vi "SNR_output.vi"() -> ()   [LabVIEW 2019]
uses:
  MeasSNRResults.ctl
  <vilib>/imath/engines/lvmath2/RunTimeEngine/Managers/WorkSpace/UID Generator.vi
  <vilib>/imath/engines/lvmath2/RunTimeEngine/RunTimeType/NIMS_RunTimeType_From StrictType (excl LVString).vi
  <instcachedir>/0/NIMS_RunTimeType_From StrictType (excl LVString)_D8AFBA86A94845AAA577C895450664BD.lvgen/NIMS_RunTimeType_From StrictType (excl LVString)_D8AFBA86A94845AAA577C895450664BD_000.vi
  <vilib>/imath/engines/lvmath2/RunTimeEngine/LocalVariableDefStatement/MC_LocalVariableDefStatement_Display.vi
  <vilib>/imath/engines/lvmath2/RunTimeEngine/Managers/SymbolTable/Clear UID.vi
  <vilib>/imath/engines/lvmath2/RunTimeEngine/NodeEndStatement/NIMS_NodeEndStatement_Output.vi
  <instcachedir>/0/NIMS_NodeEndStatement_Output_53EC0D466D134D7ABD903AC30B43404B.lvgen/NIMS_NodeEndStatement_Output_53EC0D466D134D7ABD903AC30B43404B_009.vi
  <instcachedir>/0/NIMS_NodeEndStatement_Output_53EC0D466D134D7ABD903AC30B43404B.lvgen/NIMS_NodeEndStatement_Output_53EC0D466D134D7ABD903AC30B43404B_001.vi
  <vilib>/imath/engines/lvmath2/RunTimeEngine/ErrorHandling/NIMS_Finalize Error.vi
  <vilib>/measure/NI_MABase.lvlib
  <vilib>/imath/engines/lvmath2/RunTimeEngine/Managers/SymbolTable/NIMS_WorkSpace.lvlib
panel:
  in  "Tab Control":enum32{"Part 1", "Part 2", "Part 3", "Part 4"}(tab)=enum."Part 4"
  in  "standard deviation":dbl=0.1 format="%.2p"
  in  "amplitude":dbl=1.0 format="%0.2p"
  in  "frequency":dbl=1001.0 format="%0.2p"
  in  "VRef":dbl=1.0
  in  "LowerNoiseBW":dbl
  in  "IgnoreDC":bool
  in  "sampling info":cluster{"Fs":dbl, "#s":dbl}={"Fs"=100000.0, "#s"=20000.0} {"Fs" format="%.2p"}
  out "MeasSNRResults":T1={"VSignalRMS"=0.7053309596420384, "VNoiseRMS"=0.09844196981459605, "SNR(dB)"=17.10425303559703, "NumBits"=2.548879241793527, "SNRFS(dB)"=17.12609413716782, "NumBitsFS"=2.552507331755452} {"SNRFS(dB)" format="%_3p"; "NumBitsFS" format="%.1f"; "NumBits" format="%.1f"; "SNR(dB)" format="%_3p"; "VNoiseRMS" format="%#_3p"; "VSignalRMS" format="%#_3p"}
  out "Input":waveform(dbl)(graph)={"t0"=timestamp(0 s since 1904-01-01), "dt"=1e-05, "Y"=array[20000 elements]} caption="Histogram"
  out "MeasSNR Expected":T1={"VSignalRMS"=0.7071067811865475, "VNoiseRMS"=0.1, "SNR(dB)"=16.989700043360187, "NumBits"=2.5298505055415594, "SNRFS(dB)"=16.989700043360187, "NumBitsFS"=2.8200236127281304} {"SNRFS(dB)" format="%_3p"; "NumBitsFS" format="%.1f"; "NumBits" format="%.1f"; "SNR(dB)" format="%_3p"; "VNoiseRMS" format="%#_3p"; "VSignalRMS" format="%#_3p"}
  out "UpperNoiseBW":dbl=50000.0
  out "Mag Spectrum 1":cluster{"f0":dbl, "df":dbl, "magnitude":dbl[]}(graph)={"f0"=0.0, "df"=5.0, "magnitude"=array[10000 elements]} caption="Histogram"
  in  "IgnoreDC 2":bool=TRUE
  in  "LowerNoiseBW 2":dbl
  in  "VRef 2":dbl=1.0
  in  "sampling info 2":cluster{"Fs":dbl, "#s":dbl}={"Fs"=100000.0, "#s"=20000.0} {"Fs" format="%.2p"}
  out "Input 2":waveform(dbl)(graph)={"t0"=timestamp(2.8000000000000003 s since 1904-01-01), "dt"=1e-05, "Y"=array[20000 elements]} caption="Histogram"
  in  "amplitude 2":dbl=1.0 format="%0.2p"
  in  "frequency 2":dbl=1001.0 format="%0.2p"
  out "delta":dbl=7.62939453125e-06
  out "sigma":dbl=2.2024164931855234e-06
  out "MeasSNRResults 2":T1={"VSignalRMS"=0.7071067986176297, "VNoiseRMS"=2.453932856011485e-06, "SNR(dB)"=109.19244674787093, "NumBits"=17.845921386689525, "SNRFS(dB)"=109.1924465337527, "NumBitsFS"=17.84592135112171} {"SNRFS(dB)" format="%_3p"; "NumBitsFS" format="%.1f"; "NumBits" format="%.1f"; "SNR(dB)" format="%_3p"; "VNoiseRMS" format="%#_3p"; "VSignalRMS" format="%#_3p"}
  out "2^(N-1)/Vref":dbl=131072.0
  out "Results: Bits 4-18":T1[](array[typedef])=[{"VSignalRMS"=0.7101470628693265, "VNoiseRMS"=0.038700707438026845, "SNR(dB)"=25.272587825922308, "NumBits"=3.905745486033606, "SNRFS(dB)"=25.235321965915688, "NumBitsFS"=3.899555143839815}, {"VSignalRMS"=0.7082317616189774, "VNoiseRMS"=0.019483292047133716, "SNR(dB)"=31.210261178048867, "NumBits"=4.892069963131041, "SNRFS(dB)"=31.196453233668976, "NumBitsFS"=4.889776284662621}, {"VSignalRMS"=0.7074174458063527, "VNoiseRMS"=0.009851316989764243, "SNR(dB)"=37.12362944196923, "NumBits"=5.874357050161002, "SNRFS(dB)"=37.119814168121, "NumBitsFS"=5.873723283741032}, {"VSignalRMS"=0.707070558192555, "VNoiseRMS"=0.0049426927430694465, "SNR(dB)"=43.109982802020106, "NumBits"=6.868767907312311, "SNRFS(dB)"=43.11042776591464, "NumBitsFS"=6.8688418215805065}, {"VSignalRMS"=0.7071264669443802, "VNoiseRMS"=0.0024726949970293767, "SNR(dB)"=49.12653085128376, "NumBits"=7.868194493568732, "SNRFS(dB)"=49.126289040648615, "NumBitsFS"=7.868154325689139}, {"VSignalRMS"=0.707117724944963, "VNoiseRMS"=0.0012448255565093345, "SNR(dB)"=55.08766455446092, "NumBits"=8.858416038946999, "SNRFS(dB)"=55.087530125623886, "NumBitsFS"=8.858393708575397}, {"VSignalRMS"=0.7071124254509354, "VNoiseRMS"=0.0006223588128025631, "SNR(dB)"=61.108952501973235, "NumBits"=9.858629983716485, "SNRFS(dB)"=61.10888316978296, "NumBitsFS"=9.858618466741357}, {"VSignalRMS"=0.7071037089140556, "VNoiseRMS"=0.00031251710643333074, "SNR(dB)"=67.09218641311259, "NumBits"=10.85252265998548, "SNRFS(dB)"=67.09222415207716, "NumBitsFS"=10.852528928916472}, {"VSignalRMS"=0.7071095465375292, "VNoiseRMS"=0.00015693733289259758, "SNR(dB)"=73.07520865966347, "NumBits"=11.846380176023834, "SNRFS(dB)"=73.07517469097995, "NumBitsFS"=11.846374533385374}, {"VSignalRMS"=0.7071066273851384, "VNoiseRMS"=7.82240526480512e-05, "SNR(dB)"=79.12289190974586, "NumBits"=12.850978722549145, "SNRFS(dB)"=79.12289379899688, "NumBitsFS"=12.85097903637822}, {"VSignalRMS"=0.7071071974582727, "VNoiseRMS"=3.923353200600109e-05, "SNR(dB)"=85.11655701009964, "NumBits"=13.846604154501602, "SNRFS(dB)"=85.11655189674293, "NumBitsFS"=13.8466033051068}, {"VSignalRMS"=0.7071067703059197, "VNoiseRMS"=1.9490215277495725e-05, "SNR(dB)"=91.19336718757692, "NumBits"=14.85604106105929, "SNRFS(dB)"=91.19336732123132, "NumBitsFS"=14.856041083261017}, {"VSignalRMS"=0.7071070439602097, "VNoiseRMS"=9.831535653299205e-06, "SNR(dB)"=97.13727610139594, "NumBits"=15.843401345746834, "SNRFS(dB)"=97.13727287356294, "NumBitsFS"=15.843400809561949}, {"VSignalRMS"=0.707106815641892, "VNoiseRMS"=4.877354535522192e-06, "SNR(dB)"=103.22601395339575, "NumBits"=16.854819593587333, "SNRFS(dB)"=103.22601353015655, "NumBitsFS"=16.85481952328182}, {"VSignalRMS"=0.7071067986176297, "VNoiseRMS"=2.453932856011485e-06, "SNR(dB)"=109.19244674787093, "NumBits"=17.845921386689525, "SNRFS(dB)"=109.1924465337527, "NumBitsFS"=17.84592135112171}] {"SNRFS(dB)" format="%_3p"; "NumBitsFS" format="%.1f"; "NumBits" format="%.1f"; "SNR(dB)" format="%_3p"; "VNoiseRMS" format="%#_3p"; "VSignalRMS" format="%#_3p"}
  out "Expected: Bits 4-18 2":T1[](array[typedef])=[{"VSignalRMS"=0.7071067811865475, "VNoiseRMS"=0.036084391824351615, "SNR(dB)"=25.843312243675307, "NumBits"=4.0005502065905825, "SNRFS(dB)"=25.843312243675307, "NumBitsFS"=4.0005502065905825}, {"VSignalRMS"=0.7071067811865475, "VNoiseRMS"=0.018042195912175808, "SNR(dB)"=31.86391215695493, "NumBits"=5.0006498599592915, "SNRFS(dB)"=31.86391215695493, "NumBitsFS"=5.0006498599592915}, {"VSignalRMS"=0.7071067811865475, "VNoiseRMS"=0.009021097956087904, "SNR(dB)"=37.88451207023456, "NumBits"=6.000749513328, "SNRFS(dB)"=37.88451207023456, "NumBitsFS"=6.000749513328}, {"VSignalRMS"=0.7071067811865475, "VNoiseRMS"=0.004510548978043952, "SNR(dB)"=43.90511198351418, "NumBits"=7.0008491666967085, "SNRFS(dB)"=43.90511198351418, "NumBitsFS"=7.0008491666967085}, {"VSignalRMS"=0.7071067811865475, "VNoiseRMS"=0.002255274489021976, "SNR(dB)"=49.92571189679381, "NumBits"=8.000948820065418, "SNRFS(dB)"=49.92571189679381, "NumBitsFS"=8.000948820065418}, {"VSignalRMS"=0.7071067811865475, "VNoiseRMS"=0.001127637244510988, "SNR(dB)"=55.946311810073425, "NumBits"=9.001048473434125, "SNRFS(dB)"=55.946311810073425, "NumBitsFS"=9.001048473434125}, {"VSignalRMS"=0.7071067811865475, "VNoiseRMS"=0.000563818622255494, "SNR(dB)"=61.96691172335305, "NumBits"=10.001148126802834, "SNRFS(dB)"=61.96691172335305, "NumBitsFS"=10.001148126802834}, {"VSignalRMS"=0.7071067811865475, "VNoiseRMS"=0.000281909311127747, "SNR(dB)"=67.98751163663268, "NumBits"=11.001247780171541, "SNRFS(dB)"=67.98751163663268, "NumBitsFS"=11.001247780171541}, {"VSignalRMS"=0.7071067811865475, "VNoiseRMS"=0.0001409546555638735, "SNR(dB)"=74.0081115499123, "NumBits"=12.00134743354025, "SNRFS(dB)"=74.0081115499123, "NumBitsFS"=12.00134743354025}, {"VSignalRMS"=0.7071067811865475, "VNoiseRMS"=7.047732778193675e-05, "SNR(dB)"=80.02871146319193, "NumBits"=13.001447086908957, "SNRFS(dB)"=80.02871146319193, "NumBitsFS"=13.001447086908957}, {"VSignalRMS"=0.7071067811865475, "VNoiseRMS"=3.5238663890968374e-05, "SNR(dB)"=86.04931137647155, "NumBits"=14.001546740277666, "SNRFS(dB)"=86.04931137647155, "NumBitsFS"=14.001546740277666}, {"VSignalRMS"=0.7071067811865475, "VNoiseRMS"=1.7619331945484187e-05, "SNR(dB)"=92.06991128975118, "NumBits"=15.001646393646375, "SNRFS(dB)"=92.06991128975118, "NumBitsFS"=15.001646393646375}, {"VSignalRMS"=0.7071067811865475, "VNoiseRMS"=8.809665972742094e-06, "SNR(dB)"=98.0905112030308, "NumBits"=16.001746047015082, "SNRFS(dB)"=98.0905112030308, "NumBitsFS"=16.001746047015082}, {"VSignalRMS"=0.7071067811865475, "VNoiseRMS"=4.404832986371047e-06, "SNR(dB)"=104.11111111631043, "NumBits"=17.001845700383793, "SNRFS(dB)"=104.11111111631043, "NumBitsFS"=17.001845700383793}, {"VSignalRMS"=0.7071067811865475, "VNoiseRMS"=2.2024164931855234e-06, "SNR(dB)"=110.13171102959005, "NumBits"=18.0019453537525, "SNRFS(dB)"=110.13171102959005, "NumBitsFS"=18.0019453537525}] {"SNRFS(dB)" format="%_3p"; "NumBitsFS" format="%.1f"; "NumBits" format="%.1f"; "SNR(dB)" format="%_3p"; "VNoiseRMS" format="%#_3p"; "VSignalRMS" format="%#_3p"}
  out "UpperNoiseBW 2":dbl=50000.0
  out "Mag Spectrum 2":cluster{"f0":dbl, "df":dbl, "magnitude":dbl[]}(graph)={"f0"=0.0, "df"=5.0, "magnitude"=array[10000 elements]} caption="Histogram"
  in  "LowerNoiseBW 3":dbl
  in  "VRef 3":dbl=5.0
  in  "frequency 3":dbl=1001.0 format="%0.2p"
  in  "IgnoreDC 3":bool=TRUE
  in  "sampling info 3":cluster{"Fs":dbl, "#s":dbl}={"Fs"=100000.0, "#s"=20000.0} {"Fs" format="%.2p"}
  out "MeasSNRResults 3":T1={"VSignalRMS"=3.5362111960439835, "VNoiseRMS"=0.00039855274029478027, "SNR(dB)"=78.96104790648062, "NumBits"=12.824094336624688, "SNRFS(dB)"=78.95938413973214, "NumBitsFS"=12.823817963410654} {"SNRFS(dB)" format="%_3p"; "NumBitsFS" format="%.1f"; "NumBits" format="%.1f"; "SNR(dB)" format="%_3p"; "VNoiseRMS" format="%#_3p"; "VSignalRMS" format="%#_3p"}
  out "2^(N-1)/Vref 2":dbl=819.2
  out "sigma 2":dbl=0.00035238663890968373
  out "delta 2":dbl=0.001220703125
  out "Results: Bits 4-13":T1[](array[typedef])=[{"VSignalRMS"=3.5533418214900805, "VNoiseRMS"=0.17091452154947714, "SNR(dB)"=26.35716047606195, "NumBits"=4.0859070558242445, "SNRFS(dB)"=26.313520858008555, "NumBitsFS"=4.078657949835308}, {"VSignalRMS"=3.542142802275201, "VNoiseRMS"=0.08696716973366357, "SNR(dB)"=32.19821458588856, "NumBits"=5.056181824898432, "SNRFS(dB)"=32.181993398255784, "NumBitsFS"=5.053487275457772}, {"VSignalRMS"=3.538158117160709, "VNoiseRMS"=0.04397515056705225, "SNR(dB)"=38.111398042518736, "NumBits"=6.03843821304298, "SNRFS(dB)"=38.10495342771662, "NumBitsFS"=6.0373676790226956}, {"VSignalRMS"=3.536882058385789, "VNoiseRMS"=0.02215807960508947, "SNR(dB)"=44.06176919395357, "NumBits"=7.026871959128501, "SNRFS(dB)"=44.05845776441566, "NumBitsFS"=7.026321887776688}, {"VSignalRMS"=3.536545042950174, "VNoiseRMS"=0.011106754901903125, "SNR(dB)"=50.05984011251253, "NumBits"=8.02322925457019, "SNRFS(dB)"=50.05735636631407, "NumBitsFS"=8.022816672145195}, {"VSignalRMS"=3.5362581281301697, "VNoiseRMS"=0.005588051395456805, "SNR(dB)"=56.02567133726535, "NumBits"=9.01423111914707, "SNRFS(dB)"=56.02389229340432, "NumBitsFS"=9.013935596911018}, {"VSignalRMS"=3.5361159337529484, "VNoiseRMS"=0.002784902220382939, "SNR(dB)"=62.074330875104316, "NumBits"=10.018991839718327, "SNRFS(dB)"=62.072901101419625, "NumBitsFS"=10.018754335783992}, {"VSignalRMS"=3.5362005832217522, "VNoiseRMS"=0.0014032815091866001, "SNR(dB)"=68.02784177643953, "NumBits"=11.007947138943443, "SNRFS(dB)"=68.02620407768751, "NumBitsFS"=11.00767509596138}, {"VSignalRMS"=3.5362313169756114, "VNoiseRMS"=0.0007303280743976477, "SNR(dB)"=73.70045340731076, "NumBits"=11.95024142978584, "SNRFS(dB)"=73.69874021826122, "NumBitsFS"=11.949956846887247}, {"VSignalRMS"=3.5362111960439835, "VNoiseRMS"=0.00039855274029478027, "SNR(dB)"=78.96104790648062, "NumBits"=12.824094336624688, "SNRFS(dB)"=78.95938413973214, "NumBitsFS"=12.823817963410654}] {"SNRFS(dB)" format="%_3p"; "NumBitsFS" format="%.1f"; "NumBits" format="%.1f"; "SNR(dB)" format="%_3p"; "VNoiseRMS" format="%#_3p"; "VSignalRMS" format="%#_3p"}
  out "Expected: Bits 4-13":T1[](array[typedef])=[{"VSignalRMS"=3.5355339059327373, "VNoiseRMS"=0.18042195912175807, "SNR(dB)"=25.843312243675307, "NumBits"=4.0005502065905825, "SNRFS(dB)"=25.843312243675307, "NumBitsFS"=4.0005502065905825}, {"VSignalRMS"=3.5355339059327373, "VNoiseRMS"=0.09021097956087903, "SNR(dB)"=31.86391215695493, "NumBits"=5.0006498599592915, "SNRFS(dB)"=31.86391215695493, "NumBitsFS"=5.0006498599592915}, {"VSignalRMS"=3.5355339059327373, "VNoiseRMS"=0.04510548978043952, "SNR(dB)"=37.88451207023456, "NumBits"=6.000749513328, "SNRFS(dB)"=37.88451207023456, "NumBitsFS"=6.000749513328}, {"VSignalRMS"=3.5355339059327373, "VNoiseRMS"=0.02255274489021976, "SNR(dB)"=43.90511198351418, "NumBits"=7.0008491666967085, "SNRFS(dB)"=43.90511198351418, "NumBitsFS"=7.0008491666967085}, {"VSignalRMS"=3.5355339059327373, "VNoiseRMS"=0.01127637244510988, "SNR(dB)"=49.92571189679381, "NumBits"=8.000948820065418, "SNRFS(dB)"=49.92571189679381, "NumBitsFS"=8.000948820065418}, {"VSignalRMS"=3.5355339059327373, "VNoiseRMS"=0.00563818622255494, "SNR(dB)"=55.946311810073425, "NumBits"=9.001048473434125, "SNRFS(dB)"=55.946311810073425, "NumBitsFS"=9.001048473434125}, {"VSignalRMS"=3.5355339059327373, "VNoiseRMS"=0.00281909311127747, "SNR(dB)"=61.96691172335305, "NumBits"=10.001148126802834, "SNRFS(dB)"=61.96691172335305, "NumBitsFS"=10.001148126802834}, {"VSignalRMS"=3.5355339059327373, "VNoiseRMS"=0.001409546555638735, "SNR(dB)"=67.98751163663268, "NumBits"=11.001247780171541, "SNRFS(dB)"=67.98751163663268, "NumBitsFS"=11.001247780171541}, {"VSignalRMS"=3.5355339059327373, "VNoiseRMS"=0.0007047732778193675, "SNR(dB)"=74.0081115499123, "NumBits"=12.00134743354025, "SNRFS(dB)"=74.0081115499123, "NumBitsFS"=12.00134743354025}, {"VSignalRMS"=3.5355339059327373, "VNoiseRMS"=0.00035238663890968373, "SNR(dB)"=80.02871146319193, "NumBits"=13.001447086908957, "SNRFS(dB)"=80.02871146319193, "NumBitsFS"=13.001447086908957}] {"SNRFS(dB)" format="%_3p"; "NumBitsFS" format="%.1f"; "NumBits" format="%.1f"; "SNR(dB)" format="%_3p"; "VNoiseRMS" format="%#_3p"; "VSignalRMS" format="%#_3p"}
  out "Mag Spectrum 3":cluster{"f0":dbl, "df":dbl, "magnitude":dbl[]}(graph)={"f0"=0.0, "df"=5.000000000000014, "magnitude"=array[10000 elements]} caption="Histogram"
  out "Input 3":waveform(dbl)[](graph)=[{"t0"=timestamp(1.8000000000000003 s since 1904-01-01), "dt"=1e-05, "Y"=array[20000 elements]}, {"t0"=timestamp(1.8000000000000003 s since 1904-01-01), "dt"=1e-05, "Y"=array[20000 elements]}, {"t0"=timestamp(3731601197.1711726 s since 1904-01-01), "dt"=9.999999999999972e-06, "Y"=array[20000 elements], "attributes"=variant("NI_ChannelName"=variant(string "Dev1/ai0"), "NI_UnitDescription"=variant(string "Volts"))}] caption="Histogram"
  out "UpperNoiseBW 3":dbl=50000.0
  in  "LowerNoiseBW 4":dbl
  out "UpperNoiseBW 4":dbl=9765.625
  in  "VRef 4":dbl=5.0
  in  "frequency 4":dbl=1001.0 format="%0.2p"
  in  "sampling info 4":cluster{"Fs":dbl, "#s":dbl}={"Fs"=10000000.0, "#s"=200000.0} {"Fs" format="%.2p"}
  in  "IgnoreDC 4":bool=TRUE
  out "Octave # (d)":i32=9
  out "2^d":dbl=512.0
  out "MeasSNRResults 4":T1={"VSignalRMS"=3.5355580303896903, "VNoiseRMS"=0.00013598083371339024, "SNR(dB)"=88.29960540634472, "NumBits"=14.37534973527321, "SNRFS(dB)"=88.29954613901442, "NumBitsFS"=14.375339890201731} {"SNRFS(dB)" format="%_3p"; "NumBitsFS" format="%.1f"; "NumBits" format="%.1f"; "SNR(dB)" format="%_3p"; "VNoiseRMS" format="%#_3p"; "VSignalRMS" format="%#_3p"}
  out "2^(N-1)/Vref 3":dbl=102.4
  out "QNoise (sigma)":dbl=0.00281909311127747
  out "delta 3":dbl=0.009765625
  out "Mag Spectrum 4":cluster{"f0":dbl, "df":dbl, "magnitude":dbl[]}(graph)={"f0"=0.0, "df"=50.0, "magnitude"=array[100000 elements]} caption="Histogram"
  out "Input 4":waveform(dbl)[](graph)=[{"t0"=timestamp(0.15999999999999998 s since 1904-01-01), "dt"=1e-07, "Y"=array[200000 elements]}, {"t0"=timestamp(0.15999999999999998 s since 1904-01-01), "dt"=1e-07, "Y"=array[200000 elements]}] caption="Histogram"
  out "Results: Octaves 1-8":T1[](array[typedef])=[{"VSignalRMS"=3.5355692268773713, "VNoiseRMS"=0.0022649942253767296, "SNR(dB)"=63.867844921794294, "NumBits"=10.316917761095398, "SNRFS(dB)"=63.86775814782954, "NumBitsFS"=10.31690334681554}, {"VSignalRMS"=3.5355730715293014, "VNoiseRMS"=0.0015761383889462924, "SNR(dB)"=67.01730940957434, "NumBits"=10.840084619530622, "SNRFS(dB)"=67.01721319039665, "NumBitsFS"=10.840068636278513}, {"VSignalRMS"=3.5355532975131236, "VNoiseRMS"=0.001085302747104996, "SNR(dB)"=70.25812972418623, "NumBits"=11.378426864482764, "SNRFS(dB)"=70.25808208423433, "NumBitsFS"=11.37841895086949}, {"VSignalRMS"=3.535578955947761, "VNoiseRMS"=0.0007793582998979756, "SNR(dB)"=73.13446750851037, "NumBits"=11.856223838622984, "SNRFS(dB)"=73.1343568330152, "NumBitsFS"=11.856205453989237}, {"VSignalRMS"=3.535547602797308, "VNoiseRMS"=0.0005486057349155165, "SNR(dB)"=76.18392691482983, "NumBits"=12.362778557280702, "SNRFS(dB)"=76.18389326525191, "NumBitsFS"=12.36277296764982}, {"VSignalRMS"=3.535566206247866, "VNoiseRMS"=0.0003588400713529196, "SNR(dB)"=79.87116079600936, "NumBits"=12.975275879735774, "SNRFS(dB)"=79.87108144287674, "NumBitsFS"=12.975262698152283}, {"VSignalRMS"=3.5355569462516105, "VNoiseRMS"=0.0002731568544831538, "SNR(dB)"=82.24091467417654, "NumBits"=13.368922703351585, "SNRFS(dB)"=82.2408580702745, "NumBitsFS"=13.36891330071005}, {"VSignalRMS"=3.535554606643994, "VNoiseRMS"=0.00018347461944034075, "SNR(dB)"=85.69763107486865, "NumBits"=13.943128085526354, "SNRFS(dB)"=85.69758021874006, "NumBitsFS"=13.943119637664461}, {"VSignalRMS"=3.5355580303896903, "VNoiseRMS"=0.00013598083371339024, "SNR(dB)"=88.29960540634472, "NumBits"=14.37534973527321, "SNRFS(dB)"=88.29954613901442, "NumBitsFS"=14.375339890201731}] {"SNRFS(dB)" format="%_3p"; "NumBitsFS" format="%.1f"; "NumBits" format="%.1f"; "SNR(dB)" format="%_3p"; "VNoiseRMS" format="%#_3p"; "VSignalRMS" format="%#_3p"}
  out "Expected: Octaves 1-8":T1[](array[typedef])=[{"VSignalRMS"=3.5355339059327373, "VNoiseRMS"=0.0019933998557805812, "SNR(dB)"=64.97721167999286, "NumBits"=10.501197953487187, "SNRFS(dB)"=64.97721167999286, "NumBitsFS"=10.501197953487187}, {"VSignalRMS"=3.5355339059327373, "VNoiseRMS"=0.001409546555638735, "SNR(dB)"=67.98751163663268, "NumBits"=11.001247780171541, "SNRFS(dB)"=67.98751163663268, "NumBitsFS"=11.001247780171541}, {"VSignalRMS"=3.5355339059327373, "VNoiseRMS"=0.0009966999278902906, "SNR(dB)"=70.99781159327249, "NumBits"=11.501297606855895, "SNRFS(dB)"=70.99781159327249, "NumBitsFS"=11.501297606855895}, {"VSignalRMS"=3.5355339059327373, "VNoiseRMS"=0.0007047732778193675, "SNR(dB)"=74.0081115499123, "NumBits"=12.00134743354025, "SNRFS(dB)"=74.0081115499123, "NumBitsFS"=12.00134743354025}, {"VSignalRMS"=3.5355339059327373, "VNoiseRMS"=0.0004983499639451453, "SNR(dB)"=77.01841150655211, "NumBits"=12.501397260224604, "SNRFS(dB)"=77.01841150655211, "NumBitsFS"=12.501397260224604}, {"VSignalRMS"=3.5355339059327373, "VNoiseRMS"=0.00035238663890968373, "SNR(dB)"=80.02871146319193, "NumBits"=13.001447086908957, "SNRFS(dB)"=80.02871146319193, "NumBitsFS"=13.001447086908957}, {"VSignalRMS"=3.5355339059327373, "VNoiseRMS"=0.00024917498197257266, "SNR(dB)"=83.03901141983174, "NumBits"=13.501496913593312, "SNRFS(dB)"=83.03901141983174, "NumBitsFS"=13.501496913593312}, {"VSignalRMS"=3.5355339059327373, "VNoiseRMS"=0.00017619331945484186, "SNR(dB)"=86.04931137647155, "NumBits"=14.001546740277666, "SNRFS(dB)"=86.04931137647155, "NumBitsFS"=14.001546740277666}, {"VSignalRMS"=3.5355339059327373, "VNoiseRMS"=0.00012458749098628633, "SNR(dB)"=89.05961133311136, "NumBits"=14.50159656696202, "SNRFS(dB)"=89.05961133311136, "NumBitsFS"=14.50159656696202}] {"SNRFS(dB)" format="%_3p"; "NumBitsFS" format="%.1f"; "NumBits" format="%.1f"; "SNR(dB)" format="%_3p"; "VNoiseRMS" format="%#_3p"; "VSignalRMS" format="%#_3p"}
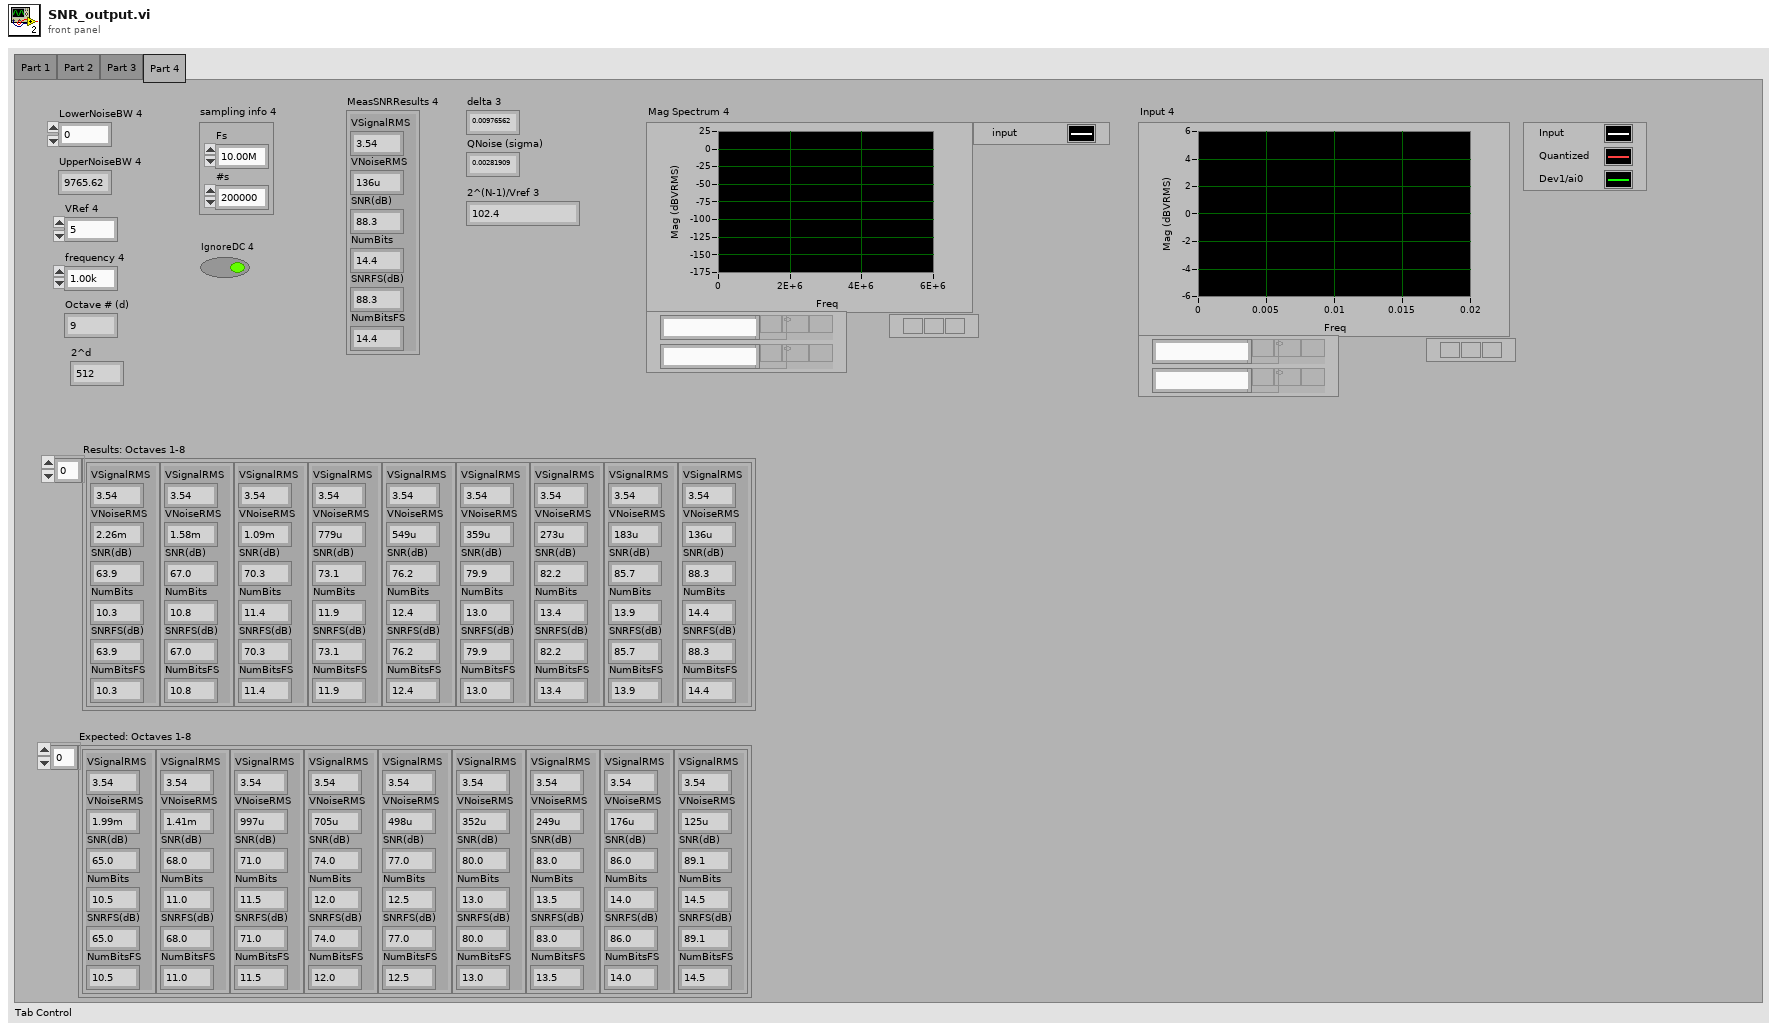
[diagram p1: front panel]
types:
  T1 = typedef "MeasSNRResults.ctl" = cluster{"VSignalRMS":dbl, "VNoiseRMS":dbl, "SNR(dB)":dbl, "NumBits":dbl, "SNRFS(dB)":dbl, "NumBitsFS":dbl}
  T2 = enum16{"Sine Wave", "Triangle Wave", "Square Wave", "Sawtooth Wave"}
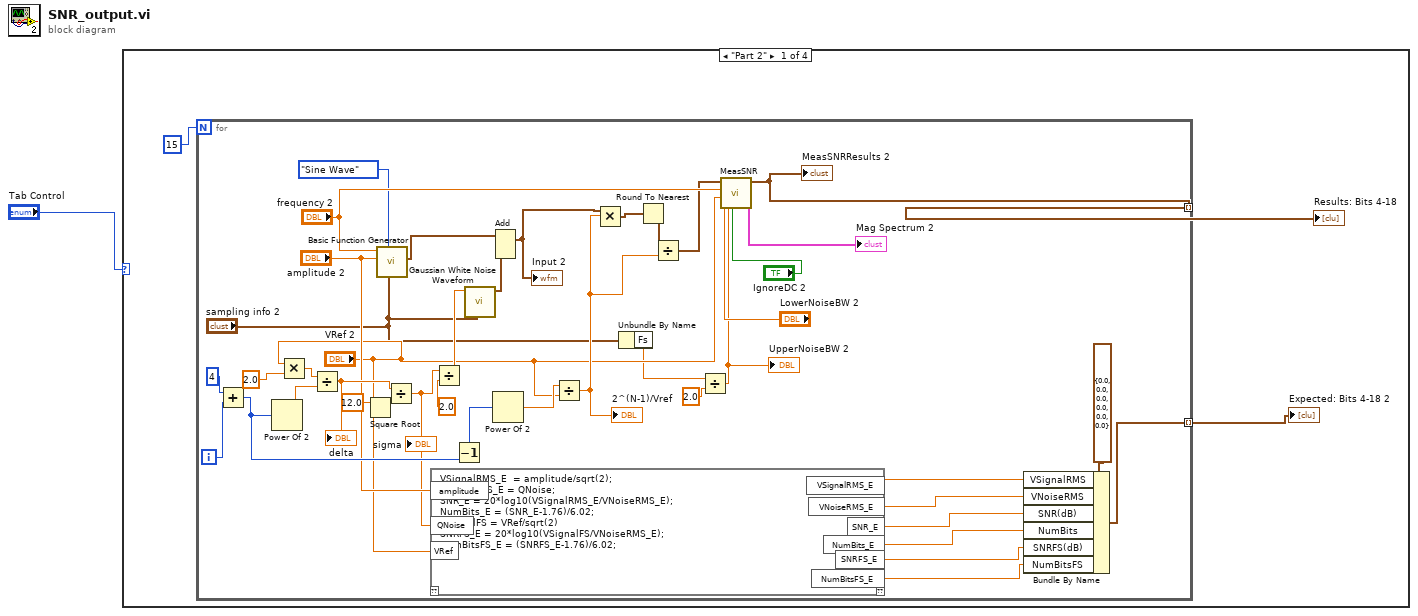
[diagram p0: block diagram]
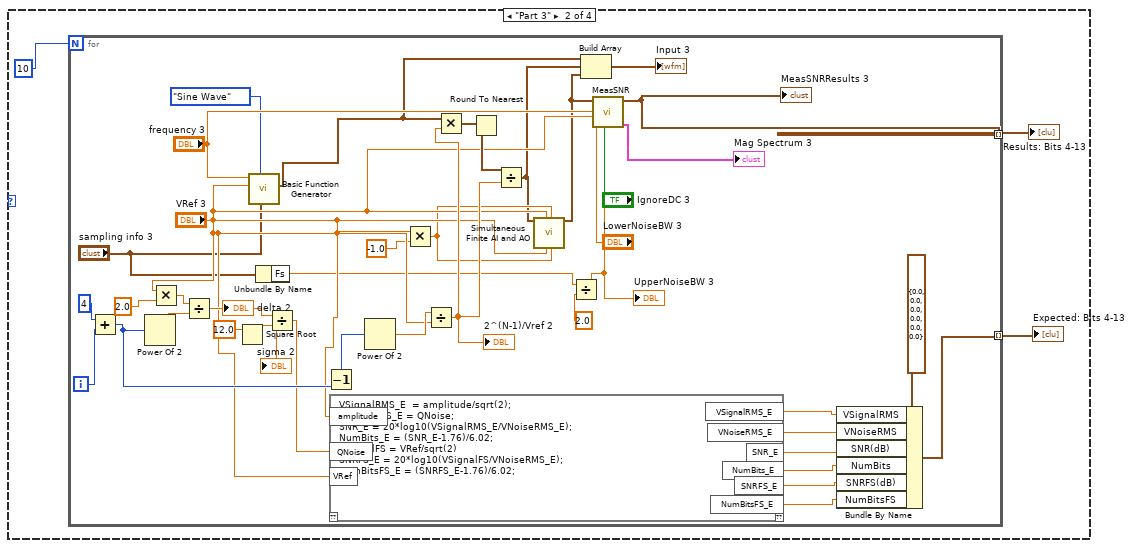
[diagram p2: hidden frame]
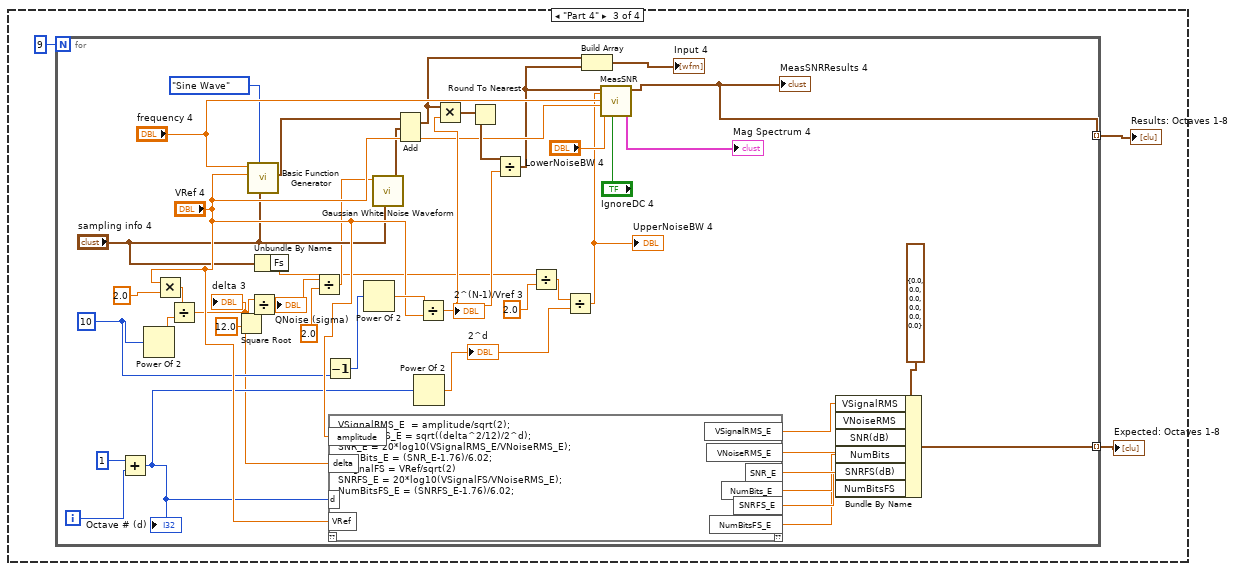
[diagram p3: hidden frame]
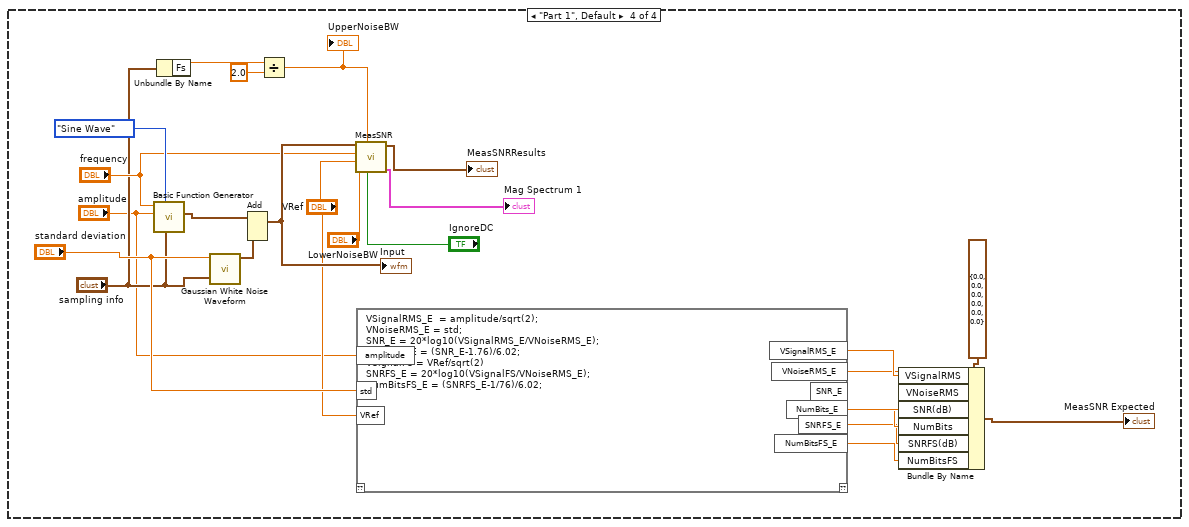
[diagram p4: hidden frame]
diagram:
  n1 = case shown="\"Part 2\"" "Tab Control" {
    frame "Part 2" {
      n2 = for {
        N: 15 -> [_]
        tunnel: [w21] -> w3 mode=indexing
        tunnel: [w10] -> w2 mode=indexing
        i -> [w39]
        n3 = Add(x=4, y=w39) -> (x+y=w22:i32)
        n4 = Power Of 2(x=w22) -> (2^x=w35:dbl)
        n5 = Multiply(x="VRef 2", y=2.0) -> (x*y=w36:dbl)
        n6 = Divide(x=w36, y=w35) -> (x/y=w34:dbl)
        "delta" <- w34
        n7 = Square Root(x=12.0) -> (sqrt(x)=w33:dbl)
        n8 = call <vilib>:"Basic Function Generator.vi"("sampling info"="sampling info 2", "signal type"=T2."Sine Wave", "amplitude"="amplitude 2", "frequency"="frequency 2") -> ("signal out"=w45:waveform(dbl))  [unwired: 5 in, 2 out]
        n9 = Divide(x=w34, y=w33) -> (x/y=w19:dbl)
        "sigma" <- w19
        n10 = mathscript code="VSignalRMS_E  = amplitude/sqrt(2);\nVNoiseRMS_E = QNoise;\nSNR_E = 20*log10(VSignalRMS_E/VNoiseRMS_E);\nNumBits_E = (SNR_E-1.76)/6.02;\nVSignalFS = VRef/sqrt(2)\nSNRFS_E = 20*log10(VSignalFS/VNoiseRMS_E);\nNumBitsFS_E = (SNRFS_E-1.76)/6.02;"("amplitude"="amplitude 2", "QNoise"=w19, "VRef"="VRef 2") -> ("VNoiseRMS_E"=w18:dbl, "SNR_E"=w16:cdb, "VSignalRMS_E"=w17:cdb, "NumBits_E"=w15:cdb, "SNRFS_E"=w13:cdb, "NumBitsFS_E"=w12:cdb)  [unwired: 1 in, 1 out]
        n11 = Divide(x=w19, y=2.0) -> (x/y=w31:dbl)
        n12 = Decrement(x=w22) -> (x-1=w28:i32)
        n13 = call <vilib>:"Gaussian White Noise Waveform.vi"("sampling info"="sampling info 2", "standard deviation"=w31) -> ("signal out"=w44:waveform(dbl))  [unwired: 8 in, 1 out]
        n14 = Add(1:w44, 2:w45) -> (0:w29:waveform(dbl))  [unwired: 1 in, 1 out]
        "Input 2" <- w29
        n15 = Power Of 2(x=w28) -> (2^x=w23:dbl)
        n16 = Divide(x=w23, y="VRef 2") -> (x/y=w27:dbl)
        "2^(N-1)/Vref" <- w27
        n17 = Multiply(x=w29, y=w27) -> (x*y=w26:waveform(dbl))
        n18 = Unbundle By Name("sampling info 2") -> ("Fs"=w8:dbl)
        n19 = Round To Nearest(number=w26) -> (nearest integer value=w25:waveform(dbl))
        n20 = Divide(x=w25, y=w27) -> (x/y=w24:waveform(dbl))
        n21 = Divide(x=w8, y=2.0) -> (x/y=w6:dbl)
        "UpperNoiseBW 2" <- w6
        n22 = call "MeasSNR.vi"("IgnoreDC"="IgnoreDC 2", "UpperNoiseBW"=w6, "LowerNoiseBW"="LowerNoiseBW 2", "VRef"="VRef 2", "FSignal"="frequency 2", "Input"=w24) -> ("Mag Spectrum"=→"Mag Spectrum 2":cluster{"f0":dbl, "df":dbl, "magnitude":dbl[]}, "MeasSNRResults"=w21:T1)  [unwired: 4 in]
        "MeasSNRResults 2" <- w21
        n23 = Bundle By Name(cluster=T1 {"VSignalRMS"=0.0, "VNoiseRMS"=0.0, "SNR(dB)"=0.0, "NumBits"=0.0, "SNRFS(dB)"=0.0, "NumBitsFS"=0.0} ("MeasSNRResults"), "VSignalRMS"=w17, "VNoiseRMS"=w18, "SNR(dB)"=w16, "NumBits"=w15, "SNRFS(dB)"=w13, "NumBitsFS"=w12) -> (w10:T1)
      }
      "Results: Bits 4-18" <- w3
      "Expected: Bits 4-18 2" <- w2
    }
    frame "Part 3" {
      n24 = for {
        N: 10 -> [_]
        tunnel: [w179] -> w157 mode=indexing
        tunnel: [w171] -> w155 mode=indexing
        i -> [w193]
        n25 = Add(x=4, y=w193) -> (x+y=w180:i32)
        n26 = Power Of 2(x=w180) -> (2^x=w189:dbl)
        n27 = Multiply(x="VRef 3", y=2.0) -> (x*y=w190:dbl)
        n28 = Divide(x=w190, y=w189) -> (x/y=w188:dbl)
        "delta 2" <- w188
        n29 = Square Root(x=12.0) -> (sqrt(x)=w187:dbl)
        n30 = call <vilib>:"Basic Function Generator.vi"("sampling info"="sampling info 3", "signal type"=T2."Sine Wave", "amplitude"="VRef 3", "frequency"="frequency 3") -> ("signal out"=w163:waveform(dbl))  [unwired: 5 in, 2 out]
        n31 = Unbundle By Name("sampling info 3") -> ("Fs"=w159:dbl)
        n32 = Divide(x=w188, y=w187) -> (x/y=w170:dbl)
        "sigma 2" <- w170
        n33 = Decrement(x=w180) -> (x-1=w185:i32)
        n34 = mathscript code="VSignalRMS_E  = amplitude/sqrt(2);\nVNoiseRMS_E = QNoise;\nSNR_E = 20*log10(VSignalRMS_E/VNoiseRMS_E);\nNumBits_E = (SNR_E-1.76)/6.02;\nVSignalFS = VRef/sqrt(2)\nSNRFS_E = 20*log10(VSignalFS/VNoiseRMS_E);\nNumBitsFS_E = (SNRFS_E-1.76)/6.02;"("amplitude"="VRef 3", "QNoise"=w170, "VRef"="VRef 3") -> ("VNoiseRMS_E"=w177:dbl, "SNR_E"=w176:cdb, "VSignalRMS_E"=w178:cdb, "NumBits_E"=w175:cdb, "SNRFS_E"=w174:cdb, "NumBitsFS_E"=w173:cdb)  [unwired: 1 in, 1 out]
        n35 = Power Of 2(x=w185) -> (2^x=w181:dbl)
        n36 = Multiply(x="VRef 3", y=-1.0) -> (x*y=w167:dbl)
        n37 = Divide(x=w181, y="VRef 3") -> (x/y=w184:dbl)
        "2^(N-1)/Vref 2" <- w184
        n38 = Multiply(x=w163, y=w184) -> (x*y=w183:waveform(dbl))
        n39 = Round To Nearest(number=w183) -> (nearest integer value=w182:waveform(dbl))
        n40 = Divide(x=w182, y=w184) -> (x/y=w164:waveform(dbl))
        n41 = call "Simultaneous Finite AI and AO.vi"("AO\nData"=w164, "AO\nVMax"="VRef 3", "AI\nVMax"="VRef 3", "AO\nVMin"=w167, "AI\nVMin"=w167) -> ("AI\nData"=w165:waveform(dbl))  [unwired: 13 in, 1 out]
        n42 = Divide(x=w159, y=2.0) -> (x/y=w158:dbl)
        "UpperNoiseBW 3" <- w158
        n43 = Build Array(w163, w164, w165) -> (→"Input 3":waveform(dbl)[])
        n44 = call "MeasSNR.vi"("IgnoreDC"="IgnoreDC 3", "UpperNoiseBW"=w158, "LowerNoiseBW"="LowerNoiseBW 3", "VRef"="VRef 3", "FSignal"="frequency 3", "Input"=w165) -> ("Mag Spectrum"=→"Mag Spectrum 3":cluster{"f0":dbl, "df":dbl, "magnitude":dbl[]}, "MeasSNRResults"=w179:T1)  [unwired: 4 in]
        "MeasSNRResults 3" <- w179
        n45 = Bundle By Name(cluster=T1 {"VSignalRMS"=0.0, "VNoiseRMS"=0.0, "SNR(dB)"=0.0, "NumBits"=0.0, "SNRFS(dB)"=0.0, "NumBitsFS"=0.0} ("MeasSNRResults"), "VSignalRMS"=w178, "VNoiseRMS"=w177, "SNR(dB)"=w176, "NumBits"=w175, "SNRFS(dB)"=w174, "NumBitsFS"=w173) -> (w171:T1)
      }
      "Results: Bits 4-13" <- w157
      "Expected: Bits 4-13" <- w155
    }
    frame "Part 4" {
      n46 = for {
        N: 9 -> [_]
        tunnel: [w327] -> w309 mode=indexing
        tunnel: [w326] -> w308 mode=indexing
        i -> [w319]
        w325 = 10 ("x")
        n47 = Add(x=1, y=w319) -> (x+y=w311:i32)
        "Octave # (d)" <- w311
        n48 = Power Of 2(x=w325) -> (2^x=w349:dbl)
        n49 = Multiply(x="VRef 4", y=2.0) -> (x*y=w350:dbl)
        n50 = Divide(x=w350, y=w349) -> (x/y=w310:dbl)
        "delta 3" <- w310
        n51 = Square Root(x=12.0) -> (sqrt(x)=w348:dbl)
        n52 = call <vilib>:"Basic Function Generator.vi"("sampling info"="sampling info 4", "signal type"=T2."Sine Wave", "amplitude"="VRef 4", "frequency"="frequency 4") -> ("signal out"=w322:waveform(dbl))  [unwired: 5 in, 2 out]
        n53 = Divide(x=w310, y=w348) -> (x/y=w336:dbl)
        "QNoise (sigma)" <- w336
        n54 = Unbundle By Name("sampling info 4") -> ("Fs"=w312:dbl)
        n55 = Divide(x=w336, y=2.0) -> (x/y=w323:dbl)
        n56 = Decrement(x=w325) -> (x-1=w347:i32)
        n57 = mathscript code="VSignalRMS_E  = amplitude/sqrt(2);\nVNoiseRMS_E = sqrt((delta^2/12)/2^d);\nSNR_E = 20*log10(VSignalRMS_E/VNoiseRMS_E);\nNumBits_E = (SNR_E-1.76)/6.02;\nVSignalFS = VRef/sqrt(2)\nSNRFS_E = 20*log10(VSignalFS/VNoiseRMS_E);\nNumBitsFS_E = (SNRFS_E-1.76)/6.02;"("amplitude"="VRef 4", "VRef"="VRef 4", "d"=w311, "delta"=w310) -> ("VNoiseRMS_E"=w341:cdb, "SNR_E"=w340:cdb, "VSignalRMS_E"=w342:cdb, "NumBits_E"=w339:cdb, "SNRFS_E"=w338:cdb, "NumBitsFS_E"=w337:cdb)  [unwired: 1 in, 1 out]
        n58 = Power Of 2(x=w347) -> (2^x=w343:dbl)
        n59 = call <vilib>:"Gaussian White Noise Waveform.vi"("sampling info"="sampling info 4", "standard deviation"=w323) -> ("signal out"=w321:waveform(dbl))  [unwired: 8 in, 1 out]
        n60 = Add(1:w321, 2:w322) -> (0:w320:waveform(dbl))  [unwired: 1 in, 1 out]
        n61 = Power Of 2(x=w311) -> (2^x=w315:dbl)
        "2^d" <- w315
        n62 = Divide(x=w343, y="VRef 4") -> (x/y=w346:dbl)
        "2^(N-1)/Vref 3" <- w346
        n63 = Multiply(x=w320, y=w346) -> (x*y=w345:waveform(dbl))
        n64 = Round To Nearest(number=w345) -> (nearest integer value=w344:waveform(dbl))
        n65 = Divide(x=w344, y=w346) -> (x/y=w314:waveform(dbl))
        n66 = Divide(x=w312, y=2.0) -> (x/y=w316:dbl)
        n67 = Divide(x=w316, y=w315) -> (x/y=w313:dbl)
        "UpperNoiseBW 4" <- w313
        n68 = Build Array(w320, w314) -> (→"Input 4":waveform(dbl)[])
        n69 = call "MeasSNR.vi"("IgnoreDC"="IgnoreDC 4", "UpperNoiseBW"=w313, "LowerNoiseBW"="LowerNoiseBW 4", "VRef"="VRef 4", "FSignal"="frequency 4", "Input"=w314) -> ("Mag Spectrum"=→"Mag Spectrum 4":cluster{"f0":dbl, "df":dbl, "magnitude":dbl[]}, "MeasSNRResults"=w326:T1)  [unwired: 4 in]
        "MeasSNRResults 4" <- w326
        n70 = Bundle By Name(cluster=T1 {"VSignalRMS"=0.0, "VNoiseRMS"=0.0, "SNR(dB)"=0.0, "NumBits"=0.0, "SNRFS(dB)"=0.0, "NumBitsFS"=0.0} ("MeasSNRResults"), "VSignalRMS"=w342, "VNoiseRMS"=w341, "SNR(dB)"=w340, "NumBits"=w339, "SNRFS(dB)"=w338, "NumBitsFS"=w337) -> (w327:T1)
      }
      "Expected: Octaves 1-8" <- w309
      "Results: Octaves 1-8" <- w308
    }
    frame "Part 1", Default {
      n71 = call <vilib>:"Basic Function Generator.vi"("sampling info"="sampling info", "signal type"=T2."Sine Wave", "amplitude"="amplitude", "frequency"="frequency") -> ("signal out"=w496:waveform(dbl))  [unwired: 5 in, 2 out]
      n72 = Unbundle By Name("sampling info") -> ("Fs"=w477:dbl)
      n73 = call <vilib>:"Gaussian White Noise Waveform.vi"("sampling info"="sampling info", "standard deviation"="standard deviation") -> ("signal out"=w495:waveform(dbl))  [unwired: 8 in, 1 out]
      n74 = Add(1:w495, 2:w496) -> (0:w493:waveform(dbl))  [unwired: 1 in, 1 out]
      "Input" <- w493
      n75 = Divide(x=w477, y=2.0) -> (x/y=w475:dbl)
      "UpperNoiseBW" <- w475
      n76 = call "MeasSNR.vi"("IgnoreDC"="IgnoreDC", "UpperNoiseBW"=w475, "LowerNoiseBW"="LowerNoiseBW", "VRef"="VRef", "FSignal"="frequency", "Input"=w493) -> ("Mag Spectrum"=→"Mag Spectrum 1":cluster{"f0":dbl, "df":dbl, "magnitude":dbl[]}, "MeasSNRResults"=→"MeasSNRResults":T1)  [unwired: 4 in]
      n77 = mathscript code="VSignalRMS_E  = amplitude/sqrt(2);\nVNoiseRMS_E = std;\nSNR_E = 20*log10(VSignalRMS_E/VNoiseRMS_E);\nNumBits_E = (SNR_E-1.76)/6.02;\nVSignalFS = VRef/sqrt(2)\nSNRFS_E = 20*log10(VSignalFS/VNoiseRMS_E);\nNumBitsFS_E = (SNRFS_E-1/76)/6.02;"("amplitude"="amplitude", "std"="standard deviation", "VRef"="VRef") -> ("VNoiseRMS_E"=w483:dbl, "SNR_E"=w482:cdb, "VSignalRMS_E"=w484:cdb, "NumBits_E"=w481:cdb, "SNRFS_E"=w480:cdb, "NumBitsFS_E"=w479:cdb)  [unwired: 1 in, 1 out]
      n78 = Bundle By Name(cluster=T1 {"VSignalRMS"=0.0, "VNoiseRMS"=0.0, "SNR(dB)"=0.0, "NumBits"=0.0, "SNRFS(dB)"=0.0, "NumBitsFS"=0.0} ("MeasSNRResults"), "VSignalRMS"=w484, "VNoiseRMS"=w483, "SNR(dB)"=w482, "NumBits"=w481, "SNRFS(dB)"=w480, "NumBitsFS"=w479) -> (→"MeasSNR Expected":T1)
    }
  }
